vi "HeartBeatDetectRealTime1.vi"() -> ()   [LabVIEW 2014, in "Phonocardiography.lvlib"]
uses:
  Phonocardiography.lvlib
  <vilib>/sound2/lvsound2.llb/Sampling Mode.ctl
  <vilib>/sound2/lvsound2.llb/Sound Data Format.ctl
  <vilib>/sound2/lvsound2.llb/Sound Input Read (DBL).vi
  <vilib>/Waveform/WDTOps.llb/WDT Get Waveform Time Array DBL.vi
  <vilib>/Analysis/NI_AAL_SigProc.lvlib
panel:
  in  "Stop":bool
  in  "Window length [s]":dbl=0.85 min=0.0 max=50.0 step=0.05
  in  "Save to":path=path "C:/Users/Tamas/Documents/Projektek/Magzati szívhang/Felvételek cikkhez/spont_1.wav"
  in  "Samples per\nLoop":i32=8192
  in  "Device ID":u32
  in  "Stop & Save":bool
  out "Heart rate":cluster{"X [s]":dbl[], "Heart Rate [BPM]":dbl[]}(graph)={"X [s]"=[1.5196833645127026, 2.3110579366474826, 3.144524522615119, 3.976732898113368, 4.747850404132086, 5.499279054881897, 6.252752154683297, 6.998049287715009, 7.786250577672999, 8.629870753148182, 9.44429067029378, 10.208377776666035, 10.9770352877609, 11.756610716914128, 12.536755242032498, 13.309895851492223, 14.120737612525563, 14.938846798465997, 15.729244360026623, 16.514211065636825, 17.259651933245834, 17.99108299053435, 18.692579761834327, 19.401293397515513, 20.217162325205646, 21.059716671717645, 21.863034308888057, 22.672384944515642, 23.450576332804726, 24.20142205426032, 24.96968823454841, 25.750915757845142, 26.534990247310358, 27.277454620017174, 28.012367962787295, 28.776510015241744, 29.560519988701692, 30.300868456933436, 30.969728914972833, 31.62839006515858, 32.3352555436007, 33.09093464054926, 33.82901862341985, 34.553171672095004, 35.305835472017826, 36.10493473491638, 36.8745361130266, 37.598383750392706, 38.347158044673606, 39.12945217697603, 39.86012600979745, 40.572897993745514, 41.38460894934675, 42.226673661017195, 42.995453308299, 43.715558803694314, 44.46819663060713, 45.19914291228759, 45.8648044263712, 46.51700546436238, 47.41442537919714, 48.31364200710193, 49.170432563913266, 49.963420096256236, 50.73540058013429, 51.47249528562212, 52.196769915861026, 52.95650798778434, 53.8580167795228, 54.777003832941766, 55.66515538564042, 56.54781293517479, 57.35617551620485, 58.18143049490885, 58.99789465121366, 59.79391868017985, 60.62286357620772, 61.52220815521514, 62.366095524850046, 63.18005746077271, 64.00618053897911, 64.80662984266834, 65.5672155221572, 66.30121962618544, 67.1042675692966, 67.96704955884377, 68.80917602217257, 69.6523766383831, 70.49114369489916, 71.30735155285502, 72.06120701191482, 72.79566612109444, 73.57107730823935, 74.38538960206857, 75.12355778439985, 75.8506535296899, 76.6523592523186, 77.47697111143235, 78.2494712067715, 79.01594987906739, 79.84678854248607, 80.67131107912847, 81.43658926865133, 82.18057197743347, 82.9913564681591, 83.77090888958094, 84.49049495316744, 85.17919060391755, 85.90285733552419, 86.65742769063915, 87.41309716625106, 88.11758089824094, 88.80565291424223, 89.54873373673023, 90.30434226488265, 91.06127178327921, 91.75875099259596, 92.449302318131, 93.12364137309997, 93.79942600255409, 94.51876953716636, 95.25838489906803, 96.04091865105504, 96.9210421244897, 97.76223492993297, 98.51494715532493, 99.20674336919255, 99.89707457955534, 100.66133803607998, 101.47099098905171, 102.23679883088856, 102.95548815809812, 103.67648221970065, 104.55065098602665, 105.42842523688307, 106.2043913337299, 106.904108130821, 107.60184290619975, 108.34032720169137, 109.12331996371951, 109.87416074352983, 110.65531292785616, 111.48468130317889, 112.2756083141637, 112.98905052612207, 113.66437010719, 114.36640808192814, 115.14219867121011, 115.95424023041613, 116.68549518229553, 117.38489581764064, 118.10889681250787, 118.85997430378421, 119.61299110764256, 120.32748028370766, 121.03182343103127, 121.86587824202508], "Heart Rate [BPM]"=[73.319264204901, 75.8174474043896, 71.98848881307141, 72.09732774448176, 77.8091529911961, 79.84790031645606, 79.63124365795504, 80.50480451458687, 76.12268688775923, 71.12205438449121, 73.67206859366814, 78.52507848858878, 78.0581717266209, 76.96497061890699, 76.90882659324731, 77.60554712282975, 73.99717538417829, 73.33984391218965, 75.91116536535242, 76.43636293256333, 80.48928172190124, 82.03097120653561, 85.53139865321258, 84.66042838632637, 73.54122453207094, 71.21202359039222, 74.69025603787641, 74.1335057499213, 77.10185553699688, 79.90989132052808, 78.0979321223026, 76.80220961340908, 76.52334160358093, 80.81195839910386, 81.64227876696462, 78.51943209679148, 76.52963869223679, 81.04291772670864, 89.70480954409462, 91.093880340566, 84.88177995654202, 79.39878215803644, 81.2915621968182, 82.85541310606993, 79.71686695461166, 75.08453928785222, 77.9624383565055, 82.89037209311682, 80.13095596133175, 76.6974946154968, 82.11598295277196, 84.17839274161442, 73.91793788905798, 71.25343120123749, 78.04577060818887, 83.32112500691558, 79.71961792846504, 82.085375497169, 90.13590049982037, 91.99617373318524, 66.85833354951502, 66.7247447812461, 70.02878302405486, 75.66323246309224, 77.72217206656478, 81.4006660925485, 82.84150444453424, 78.97458639673926, 66.55509136444115, 65.289276684343, 67.55603795060625, 67.97653295057839, 74.22411849339275, 72.70480221061526, 73.4876106154502, 75.37460907797377, 72.38116826282106, 66.71525175169265, 71.09953550549997, 73.71352068446207, 72.62840317966456, 74.95790142294177, 78.88657598749751, 81.7434121563048, 74.71533986818912, 69.54248086644775, 71.2482063119466, 71.1574432543093, 71.53356767398391, 73.51068654284481, 79.59085429298597, 81.69277125178382, 77.37830069349647, 73.68180543837342, 81.28228964097086, 82.52008128044486, 74.8404287339576, 72.76150510918589, 77.6698933268842, 78.28006462368695, 72.21618665784806, 72.7693875346696, 78.40286162788613, 80.6470355987395, 74.00240222442108, 76.96724216514507, 83.38127019991562, 87.1212123013263, 82.91109343494566, 79.51544821934935, 79.39979307939423, 85.1687516339437, 87.20017469782972, 80.74491789346266, 79.40619747464888, 79.26761810941237, 86.0240695328763, 86.88709699240955, 88.9760122269073, 88.78568316723461, 83.40938246194098, 81.12324742110594, 76.67400907328086, 68.17225288384952, 71.3272862199323, 79.71173839877011, 86.73074353003256, 86.91480132915991, 78.5069592007441, 74.10582494608015, 78.34863620106789, 83.4853082248497, 83.21843853559677, 68.63663209127276, 68.35470502974967, 77.322965840663, 85.74897765701103, 85.99256066523337, 81.2474962112192, 76.62906084161652, 79.91041724606059, 76.80961687605634, 72.34421010645886, 75.86035015455026, 84.09931315292202, 88.84682405494344, 85.46546221004554, 77.34045866105818, 73.88784394072796, 82.05072642010074, 85.78774019899687, 82.87281429910662, 79.88523247852713, 79.67949678223526, 83.9760797083553, 85.18575104761092, 71.93771825200301]}
  out "pNN50 [%]":dbl=10.897435897435898 format="%0.2f"
  out "rMSSD  [ms]":dbl=49.81776654749001 format="%0.2f"
  out "sdRR [ms]":dbl=56.15291692832544 format="%0.2f"
  out "Mean RR [ms]":dbl=771.7486222638828 format="%0.2f"
  out "Mean heart rate [BPM]":dbl=77.74552265994755
  out "Peaks":cluster{dbl[], "Amplitudes":dbl[]}[](graph)=[{array[1351680 elements], "Amplitudes"=array[1351680 elements]}, {[0.7013445465954693, 1.5196833645127026, 2.3110579366474826, 3.144524522615119, 3.976732898113368, 4.747850404132086, 5.499279054881897, 6.252752154683297, 6.998049287715009, 7.786250577672999, 8.629870753148182, 9.44429067029378, 10.208377776666035, 10.9770352877609, 11.756610716914128, 12.536755242032498, 13.309895851492223, 14.120737612525563, 14.938846798465997, 15.729244360026623, 16.514211065636825, 17.259651933245834, 17.99108299053435, 18.692579761834327, 19.401293397515513, 20.217162325205646, 21.059716671717645, 21.863034308888057, 22.672384944515642, 23.450576332804726, 24.20142205426032, 24.96968823454841, 25.750915757845142, 26.534990247310358, 27.277454620017174, 28.012367962787295, 28.776510015241744, 29.560519988701692, 30.300868456933436, 30.969728914972833, 31.62839006515858, 32.3352555436007, 33.09093464054926, 33.82901862341985, 34.553171672095004, 35.305835472017826, 36.10493473491638, 36.8745361130266, 37.598383750392706, 38.347158044673606, 39.12945217697603, 39.86012600979745, 40.572897993745514, 41.38460894934675, 42.226673661017195, 42.995453308299, 43.715558803694314, 44.46819663060713, 45.19914291228759, 45.8648044263712, 46.51700546436238, 47.41442537919714, 48.31364200710193, 49.170432563913266, 49.963420096256236, 50.73540058013429, 51.47249528562212, 52.196769915861026, 52.95650798778434, 53.8580167795228, 54.777003832941766, 55.66515538564042, 56.54781293517479, 57.35617551620485, 58.18143049490885, 58.99789465121366, 59.79391868017985, 60.62286357620772, 61.52220815521514, 62.366095524850046, 63.18005746077271, 64.00618053897911, 64.80662984266834, 65.5672155221572, 66.30121962618544, 67.1042675692966, 67.96704955884377, 68.80917602217257, 69.6523766383831, 70.49114369489916, 71.30735155285502, 72.06120701191482, 72.79566612109444, 73.57107730823935, 74.38538960206857, 75.12355778439985, 75.8506535296899, 76.6523592523186, 77.47697111143235, 78.2494712067715, 79.01594987906739, 79.84678854248607, 80.67131107912847, 81.43658926865133, 82.18057197743347, 82.9913564681591, 83.77090888958094, 84.49049495316744, 85.17919060391755, 85.90285733552419, 86.65742769063915, 87.41309716625106, 88.11758089824094, 88.80565291424223, 89.54873373673023, 90.30434226488265, 91.06127178327921, 91.75875099259596, 92.449302318131, 93.12364137309997, 93.79942600255409, 94.51876953716636, 95.25838489906803, 96.04091865105504, 96.9210421244897, 97.76223492993297, 98.51494715532493, 99.20674336919255, 99.89707457955534, 100.66133803607998, 101.47099098905171, 102.23679883088856, 102.95548815809812, 103.67648221970065, 104.55065098602665, 105.42842523688307, 106.2043913337299, 106.904108130821, 107.60184290619975, 108.34032720169137, 109.12331996371951, 109.87416074352983, 110.65531292785616, 111.48468130317889, 112.2756083141637, 112.98905052612207, 113.66437010719, 114.36640808192814, 115.14219867121011, 115.95424023041613, 116.68549518229553, 117.38489581764064, 118.10889681250787, 118.85997430378421, 119.61299110764256, 120.32748028370766, 121.03182343103127, 121.86587824202508], "Amplitudes"=[0.33165296428501273, 0.3004180439353789, 0.3185312922777503, 0.3052601169969948, 0.2753219394971568, 0.3124915060500549, 0.29155358709819673, 0.29883740695603117, 0.3008356814419773, 0.32295222947366586, 0.32183943272537896, 0.2577099302582917, 0.3075153402422978, 0.3012003112984132, 0.32306025890936974, 0.2953574212130992, 0.3353709446738182, 0.30974775036203267, 0.30092056751081414, 0.32651373446009263, 0.2980328612169978, 0.3000656208391686, 0.2616913848791655, 0.3249181168297525, 0.32846559770140166, 0.3242806372949827, 0.2939864101976182, 0.32437945980131394, 0.29180584856307185, 0.2897657711945695, 0.3097282384711384, 0.3067665730482526, 0.2847757566698311, 0.26867062768356903, 0.3324217588681113, 0.3042604631623089, 0.2740172658342943, 0.27626922736624476, 0.2697894885940621, 0.305871643567633, 0.31647054312148976, 0.31628787314582224, 0.2947127057526444, 0.2711674189070898, 0.3478736619256684, 0.3023914922547282, 0.3077427034796248, 0.30464328169361105, 0.3418417542095546, 0.3148536930631605, 0.2916710444931097, 0.3023501906810985, 0.2987978206157448, 0.32436750147019244, 0.29300697017016797, 0.2493056356042191, 0.34442658073817883, 0.29756438731966484, 0.3114212380936057, 0.27761154543692174, 0.3078936267742388, 0.3255198501909098, 0.3027061020963819, 0.2920292709813668, 0.33703558640050973, 0.3003496631066136, 0.258079320252051, 0.3083078413552056, 0.32209095822238054, 0.3496832719380831, 0.29159435081777413, 0.30937119036111765, 0.2835525640665855, 0.2786491723254403, 0.3052855923293393, 0.2535087167486557, 0.2934411250527595, 0.2982573068944507, 0.3199026695412802, 0.2731267983768498, 0.32515173071373954, 0.31185972801619055, 0.2607092357315544, 0.28299276271288504, 0.3360381543386958, 0.3012840108607273, 0.29887987059095295, 0.29931265985607686, 0.31391135652520796, 0.2936279265880782, 0.26285885023032984, 0.3005268941545282, 0.33021249656617235, 0.32371997038651984, 0.27248967530102014, 0.3327618934823753, 0.3209539313743082, 0.3156226293340531, 0.27235401763194367, 0.3204770479565513, 0.33265960414376927, 0.3268817375761947, 0.3658138073509878, 0.3064150454667494, 0.33332680472921555, 0.3156134595774387, 0.2930303182014187, 0.31550911261723275, 0.35817097522324504, 0.33040281394380844, 0.3064232223789755, 0.32054861085634884, 0.28102024736491793, 0.37200330330124864, 0.3388723368935847, 0.3170678598822018, 0.28106089094047976, 0.35489865243088203, 0.3341102873134194, 0.3253032160891651, 0.3385391837715337, 0.3128509158846898, 0.37562731221920576, 0.3627348941110659, 0.3508402130336391, 0.28483808932705135, 0.3144808656377633, 0.3512974116638325, 0.31824203573629445, 0.32045289599221805, 0.31997825035179256, 0.29997386753338345, 0.3643834490762391, 0.37557662163518474, 0.3467685963213558, 0.31689658761808953, 0.2943179810056993, 0.3416765432013399, 0.3292324858801851, 0.31333064762550067, 0.30698653628535844, 0.37861616697676714, 0.33759653613947654, 0.29024916669881173, 0.27851313018626733, 0.32195222294444825, 0.37036101228711144, 0.3402531472342048, 0.31898591791935466, 0.30518717975750154, 0.34693307101939796, 0.3431833916650554, 0.3315743870390092, 0.3125874750586787, 0.3017412165458041, 0.31497708711258937, 0.3611836825361032, 0.3433153612277492]}]
  in  "Threshold mult":dbl=0.8 min=-1.0 max=1.0 step=0.05
  in  "width (threshold)":i32=200
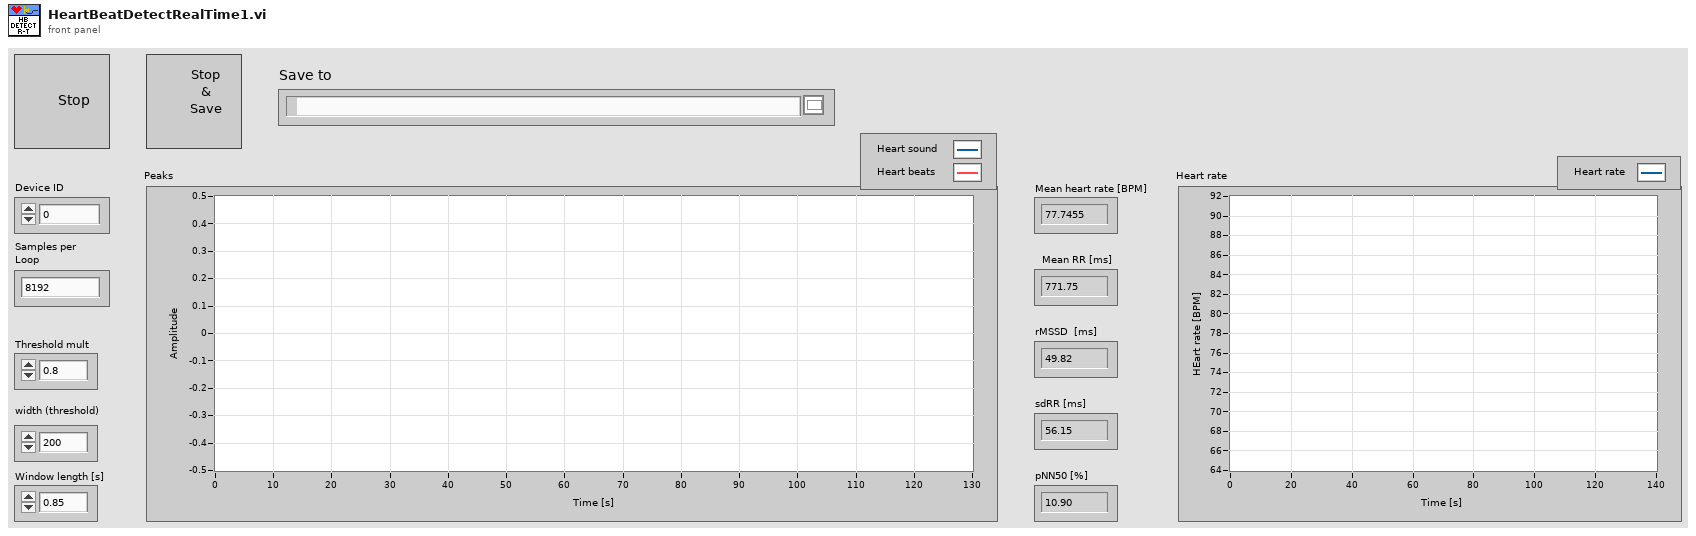
[diagram p1: front panel]
types:
  T1 = typedef "Sound Data Format.ctl" = cluster{"sample rate (S/s)":dbl, "number of channels":i32, "bits per sample":i32}
  T2 = typedef "Sampling Mode.ctl" = i32
  T3 = typedef "Sound Input Task ID.ctl" = u32
  T4 = typedef "LVCursorListTypeDef.ctl" = cluster{"Name":string, "Color":u32, "Style":u8, "Point Style":u8, "Name Visible":bool, "Allow Drag":bool, "Cursor Mode":u32, "Plot":i32, "Index":i32, "Position":cluster{"X":dbl, "Y":dbl}, "X Scale":u32, "Y Scale":u32, "Watch Plots":i32[], "Watch All Plots":bool, "Plot Area":i32, "Label Offset":cluster{"X":dbl, "Y":dbl}}[]
  T5 = cluster{"Name":string, "Color":u32, "Style":u8, "Point Style":u8, "Name Visible":bool, "Allow Drag":bool, "Cursor Mode":u32, "Plot":i32, "Index":i32, "Position":cluster{"X":dbl, "Y":dbl}, "X Scale":u32, "Y Scale":u32, "Watch Plots":i32[], "Watch All Plots":bool, "Plot Area":i32, "Label Offset":cluster{"X":dbl, "Y":dbl}}
  T6 = cluster{"Name":string, "Color":u32, "Style":u8, "Point Style":u8, "Name Visible":bool, "Allow Drag":bool, "Cursor Mode":u32, "Plot":i32, "Index":i32, "Position":cluster{"X":dbl, "Y":dbl}, "X Scale":u32, "Y Scale":u32, "Watch Plots":i32[], "Watch All Plots":bool, "Plot Area":i32, "Label Offset":cluster{"X":dbl, "Y":dbl}}[]
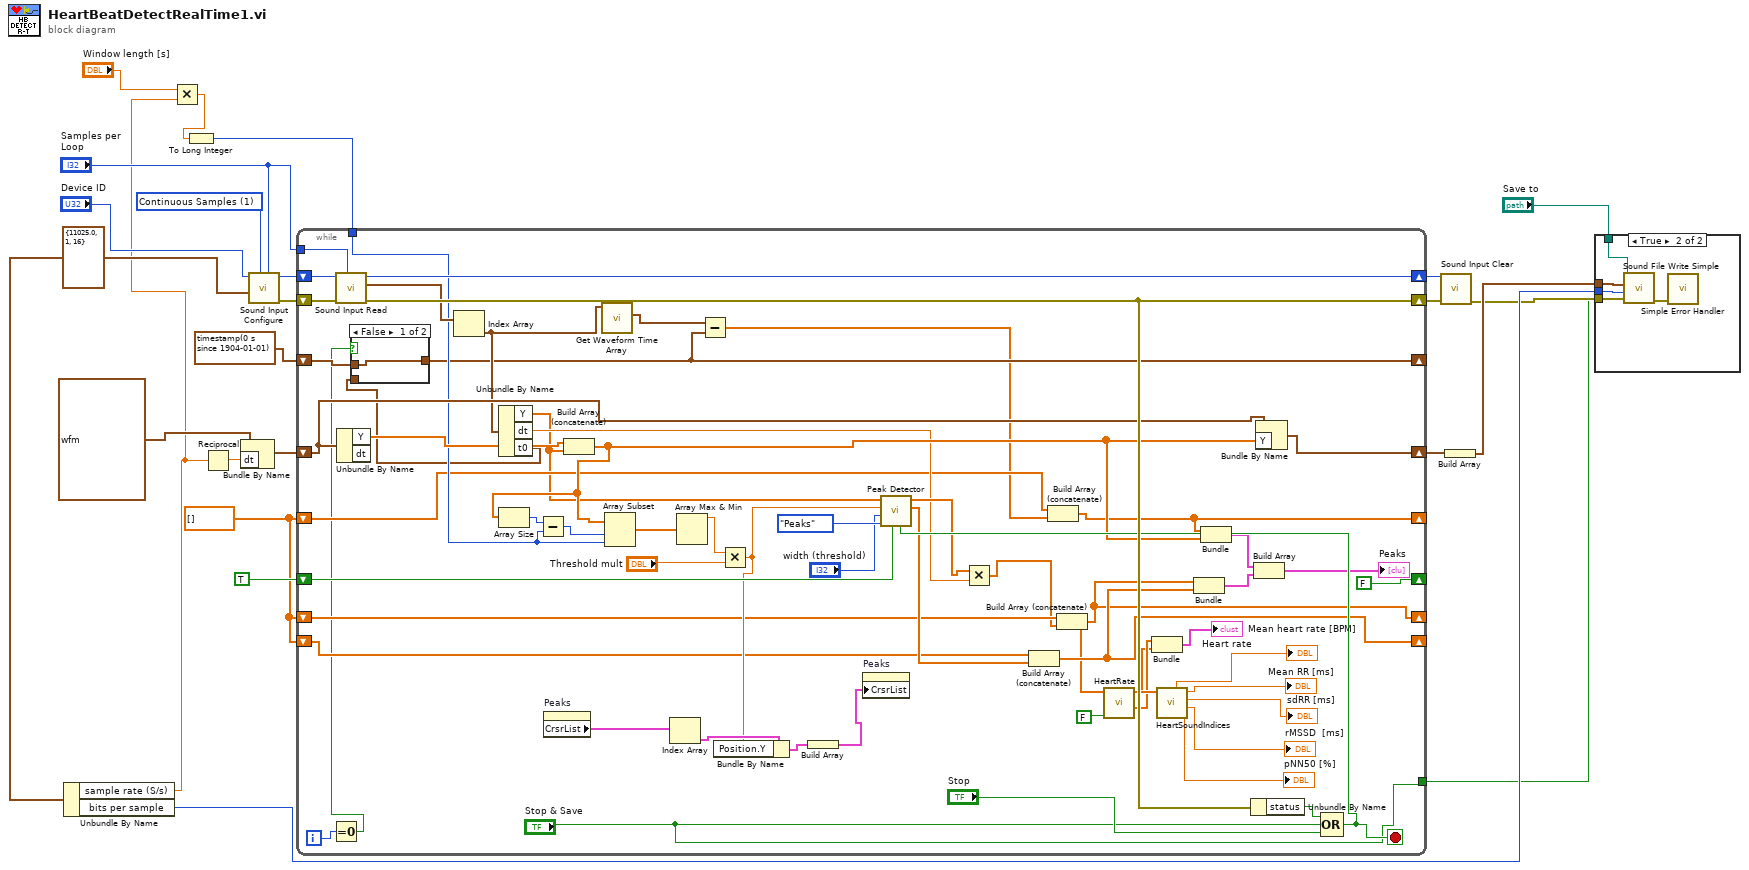
[diagram p0: block diagram]
diagram:
  w3 = dbl[] []
  w17 = T1 {"sample rate (S/s)"=11025.0, "number of channels"=1, "bits per sample"=16} ("Sound Format")
  w24 = T2 1 items=["Finite Samples", "Continuous Samples"] ("sample mode")
  n1 = Unbundle By Name(w17) -> ("sample rate (S/s)"=w7:dbl, "bits per sample"=w15:i32)
  n2 = Multiply(x="Window length [s]", y=w7) -> (x*y=w6:dbl)
  n3 = To Long Integer(number=w6) -> (32bit integer=w5:i32)
  n4 = Reciprocal(x=w7) -> (1/x=w12:dbl)
  n5 = Bundle By Name(cluster=waveform(dbl) {"t0"=timestamp(0 s since 1904-01-01), "dt"=1.0, "Y"=[]} ("element"), "dt"=w12) -> (w11:waveform(dbl))
  n6 = call <vilib>:"Sound Input Configure.vi"("number of samples/ch"="Samples per\nLoop", "sample mode"=w24, "sound format"=w17, "device ID"="Device ID") -> ("error out"=w20:errorcluster, "task ID"=w21:T3)  [unwired: 6 in]
  n7 = while {
    tunnel: "Samples per\nLoop" -> [w82]
    shift-right: [w83] -> w22
    shift-left: w21 -> [w84]
    shift-right: [w81] -> w23
    shift-left: w20 -> [w85]
    shift-right: [w77] -> w14
    shift-left: w11 -> [w78]
    tunnel: w5 -> [w74]
    shift-right: [FALSE] -> _
    shift-left: TRUE -> [w69]
    shift-right: [w40] -> _
    shift-left: w3 -> [w41]
    shift-right: [w32] -> _
    shift-left: w3 -> [w43]
    shift-right: [w42] -> _
    shift-left: w3 -> [w44]
    shift-right: [w34] -> _
    shift-left: timestamp(0 s since 1904-01-01) ("t0") -> [w38]
    tunnel: ["Stop & Save"] -> w1
    i -> [w37]
    stop <- w67 stop-if-true
    n8 = Equal To 0?(x=w37) -> (x = 0?=w36:bool)
    n9 = call-poly <vilib>:"Sound Input Read.vi"("number of samples/ch"=w82, "error in (no error)"=w85, "task ID"=w84) -> ("error out"=w81:errorcluster, "data"=w80:waveform(dbl)[], "task ID out"=w83:T3)  [unwired: 6 in]
    n10 = Unbundle By Name(w78) -> ("Y"=w79:dbl[])  [unwired: 1 out]
    n11 = Index Array(array=w80) -> (element=w47:waveform(dbl))  [unwired: 1 in]
    n12 = Unbundle By Name(w47) -> ("Y"=w25:dbl[], "dt"=w46:dbl, "t0"=w35:timestamp)
    n13 = case shown="False" w36 {
      tunnel: w38 -> [w86 _]
      tunnel: w35 -> [_ w87]
      tunnel: [w86 w87] -> w34
      frame False {
      }
      frame True {
      }
    }
    n14 = property on="Peaks" class="XYGraph (strict)"() -> ("CrsrList"=w63:T4)  [unwired: 2 in, 2 out]
    n15 = Build Array (concatenate)(w79, w25) -> (w48:dbl[])
    n16 = Array Size(array=w48) -> (size(s)=w75:i32)
    n17 = Subtract(x=w75, y=w74) -> (x-y=w73:i32)
    n18 = call-poly <vilib>:"Get Waveform Time Array.vi"("waveform in"=w47) -> ("X array"=w51:timestamp[])  [unwired: 9 in, 1 out]
    n19 = Array Subset(array=w48, index=w73, length=w74) -> (w72:dbl[])
    n20 = Index Array(array=w63) -> (element=w64:T5)  [unwired: 1 in]
    n21 = Array Max & Min(array=w72) -> (max value=w71:dbl)  [unwired: 3 out]
    n22 = Subtract(x=w51, y=w34) -> (x-y=w27:dbl[])
    n23 = Multiply(x=w71, y="Threshold mult") -> (x*y=w62:dbl)
    n24 = Bundle By Name(cluster=w64, "Position.Y"=w62) -> (w65:T5)
    n25 = Build Array(w65) -> (w66:T6)
    n26 = property on="Peaks" class="XYGraph (strict)"("CrsrList"=w66) -> ()  [unwired: 2 in, 2 out]
    n27 = Build Array (concatenate)(w41, w27) -> (w40:dbl[])
    n28 = Bundle(w40, w48) -> (w52:cluster{dbl[], dbl[]})  [unwired: 1 in]
    n29 = Unbundle By Name(w81) -> ("status"=w76:bool)
    n30 = Bundle By Name(cluster=w78, "Y"=w48) -> (w77:waveform(dbl))
    n31 = Compound Arithmetic op=OR(w76, "Stop & Save", "Stop") -> (w67:bool)
    n32 = call <vilib>:"Peak Detector.vi"("end of data (T)"=w67, "initialize (T)"=w69, "peaks/valleys"=enum32{"Peaks", "Valleys"}."Peaks", "width"="width (threshold)", "threshold"=w62, "X"=w25) -> ("Amplitudes"=w45:dbl[], "Locations"=w49:dbl[])  [unwired: 1 in, 3 out]
    n33 = Multiply(x=w49, y=w46) -> (x*y=w26:dbl[])
    n34 = Build Array (concatenate)(w44, w45) -> (w42:dbl[])
    n35 = Build Array (concatenate)(w43, w26) -> (w32:dbl[])
    n36 = call "HeartRate.vi"("Remove Ectopic?"=FALSE, "Peaks X in"=w32) -> ("X [s]"=w54:dbl[], "RR intervals [ms]"=w55:dbl[], "Heart Rate [BPM]"=w53:dbl[])  [unwired: 7 in]
    n37 = Bundle("X [s]"=w54, "Heart Rate [BPM]"=w53) -> (→"Heart rate":cluster{"X [s]":dbl[], "Heart Rate [BPM]":dbl[]})  [unwired: 1 in]
    n38 = call "HeartSoundIndices.vi"("RR intervals [ms]"=w55) -> ("pNN50 [%]"=→"pNN50 [%]":dbl, "rMSSD  [ms]"=→"rMSSD  [ms]":dbl, "sdRR [ms]"=→"sdRR [ms]":dbl, "Mean RR [ms]"=→"Mean RR [ms]":dbl, "Mean heart rate [BPM]"=→"Mean heart rate [BPM]":dbl)  [unwired: 6 in]
    n39 = Bundle(w32, w42) -> (w33:cluster{dbl[], dbl[]})  [unwired: 1 in]
    n40 = Build Array(w52, w33) -> (→"Peaks":cluster{dbl[], dbl[]}[])
  }
  n41 = call <vilib>:"Sound Input Clear.vi"("error in (no error)"=w23, "task ID"=w22) -> ("error out"=w9:errorcluster)  [unwired: 9 in]
  n42 = Build Array(w14) -> (w16:waveform(dbl)[])
  n43 = case shown="True" w1 {
    tunnel: w16 -> [_ w92]
    tunnel: w15 -> [_ w91]
    tunnel: "Save to" -> [_ w89]
    tunnel: w9 -> [_ w88]
    frame False {
    }
    frame True {
      n44 = call <vilib>:"Sound File Write Simple.vi"("error in (no error)"=w88, "bits per sample"=w91, "data"=w92, "path"=w89) -> ("error out"=w90:errorcluster)  [unwired: 6 in, 1 out]
      n45 = call <vilib>:"Simple Error Handler.vi"("error in (no error)"=w90) -> ()  [unwired: 4 in, 5 out]
    }
  }
